vi "HFRR ADV v039 new software.vi"() -> ()   [LabVIEW 2025] (continued)
            n3064 = local read "TITTLE"() -> (w3921:string)
            n3065 = call-poly <vilib>:"Append Report Text.vi"("report in"=w3946, "error in (no error)"=w3945) -> ("report out"=w3967:refnum<class "NI_report.lvclass">, "error out"=w3965:errorcluster)  [unwired: 10 in, 2 out]
            n3066 = Concatenate Strings(w3921, w3920, w3919) -> (→"output":string)
            n3067 = call-poly <vilib>:"Append Report Text.vi"("report in"=w3967, "text"=w3920, "error in (no error)"=w3965) -> ("report out"=w3966:refnum<class "NI_report.lvclass">, "error out"=w3964:errorcluster)  [unwired: 9 in, 2 out]
            n3068 = call-dynamic "Print Report.vi"("report in"=w3966, "printer name (default)"=w3974, "error in (no error)"=w3964) -> ("report out"=w3976:refnum<class "NI_report.lvclass">, "error out"=w3977:errorcluster)  [unwired: 11 in]
            n3069 = call-dynamic "Dispose Report.vi"("report in"=w3976, "error in (no error)"=w3977) -> ()  [unwired: 13 in, 1 out]
          }
        }
      }
    }
    n3070 = case shown="True" "Prog Uno" {
      frame False {
      }
      frame True {
        n3071 = stacked-sequence {
          frame #0 {
            n3072 = Delete(path (use dialog)=path "C:/LAB-IQ-NXT/UNOCOMPILE.bat" ("working directory")) -> ()  [unwired: 4 in, 3 out]
          }
          frame #1 {
            n3073 = local read "Com Port 1"() -> (w2694:refnum<visa-resource-name>)
            n3074 = Concatenate Strings("cmd.exe /c \"mode " ("command line"), w2694, ":1200,n,8,1\"\n" ("command line")) -> (w2699:string)
            n3075 = Concatenate Strings(w2699, "CD\\\nCD WinDucom\navrdude -C avrdude.conf -v -patmega328p -carduino -P" ("command line"), w2694, " -b115200 -D -Uflash:w:UNO_V20.hex:i\n" ("command line"), "\r") -> (w2701:string)
            "STR" <- w2701
            n3076 = call <vilib>:"Write Characters To File.vi"("append to file? (new file:F)"=FALSE, "character string"=w2701, "file path (dialog if empty)"=path "C:/LAB-IQ/UNOCOMPILE.bat" ("working directory")) -> ()  [unwired: 2 in, 1 out]
          }
          frame #2 {
            n3077 = disable-structure shown="Disabled" {
              frame Disabled {
                w2705 = "cmd.exe  /c \"C:\\LAB-IQ-NXT\\UNOCOMPILE.bat\"" ("string")
                n3078 = local write "Prog Uno"(FALSE ("run minimized? (F)")) -> ()
                n3079 = call <vilib>:"System Exec.vi"("expected output size  (4096)"=u32 65535, "run minimized? (F)"=FALSE, "wait until completion? (T)"=TRUE ("run minimized? (F)"), "working directory"=path "C:/LAB-IQ-NXT", "standard input"=w2705, "command line"=w2705) -> ("error out"=w2704:errorcluster, "standard output"=→"String 42":string)  [unwired: 2 in, 2 out]
                "error out 3" <- w2704
                n3080 = flat-sequence {
                  tunnel: w2704 -> [_]
                  frame #0 {
                  }
                }
              }
              frame Enabled {
              }
            }
          }
        }
      }
    }
    n3081 = Wait (ms)(milliseconds to wait=u32 50) -> ()  [unwired: 1 out]
    n3082 = Wait (ms)(milliseconds to wait=u32 50) -> ()  [unwired: 1 out]
    n3083 = local read "Quit"() -> (w2223:bool)
  }
  n3084 = while {
    stop <- w4041 stop-if-true
    n3085 = local read "Auto Start Test"() -> (w4039:bool)
    n3086 = local read "RUN"() -> (w4038:bool)
    n3087 = Wait (ms)(milliseconds to wait=u32 1000) -> ()  [unwired: 1 out]
    n3088 = Or(x=w4038, y=w4039) -> (x .or. y?=w4037:bool)
    n3089 = case shown="True" w4037 {
      frame False {
      }
      frame True {
        n3090 = local read "LVDT STROKE Actual"() -> (w4042:dbl)
        n3091 = In Range and Coerce(upper limit=1.2, x=w4042, lower limit=0.6) -> (In Range?=w4045:bool)  [unwired: 1 out]
        n3092 = call-poly <vilib>:"Random Number (Range).vi"("lower bound (0)"=0.998 ("upper bound (100)"), "upper bound (100)"=1.003) -> ("number"=w4043:dbl)  [unwired: 9 in]
        n3093 = case shown="True" w4045 {
          tunnel: [w4050 w4051] -> w4044
          tunnel: w4043 -> [_ w4051]
          tunnel: w4042 -> [w4050 _]
          frame False {
          }
          frame True {
          }
        }
        "LVDT STROKE DISPLAY" <- w4044
      }
    }
    n3094 = local read "Quit"() -> (w4041:bool)
  }
  n3095 = while {
    tunnel: [w4068] -> w49
    shift-right: [w4061] -> _
    shift-left: 0.0 -> [w4064]
    shift-right: [w4060] -> _
    shift-left: 0.0 -> [w4063]
    shift-right: [w4059] -> _
    shift-left: 100.0 ("vc_cmd") -> [w4062]
    stop <- w4068 stop-if-true
    # "PID LOGIC"
    n3096 = local read "run test Calibration"() -> (w4056:bool)
    n3097 = local read "RUN"() -> (w4066:bool)
    n3098 = local read "Auto Start Temp"() -> (w4057:bool)
    n3099 = local read "Auto Start Test"() -> (w4065:bool)
    n3100 = local read "START TEMP"() -> (w4055:bool)
    n3101 = And(x=w4057, y=w4065) -> (x .and. y?=w4058:bool)
    n3102 = Or(x=w4066, y=w4058) -> (x .or. y?=w4067:bool)
    n3103 = And(x=w4067, y=w4055) -> (x .and. y?=w4054:bool)
    n3104 = And(x=w4056, y=w4055) -> (x .and. y?=w4053:bool)
    n3105 = Or(x=w4053, y=w4054) -> (x .or. y?=w4052:bool)
    n3106 = Wait (ms)(milliseconds to wait="milliseconds to wait") -> ()  [unwired: 1 out]
    n3107 = case shown="True" w4052 {
      tunnel: [400.0 ("out_vc_cmd") w4087] -> w4059
      tunnel: [w4071 w4089] -> w4060
      tunnel: [w4071 w4088] -> w4061
      tunnel: w4064 -> [_ w4078]
      tunnel: w4063 -> [_ w4077]
      tunnel: w4062 -> [_ w4076]
      tunnel: w4056 -> [_ w4072]
      frame False {
        w4071 = 0.0 ("error_out")
      }
      frame True {
        n3108 = case shown="True" w4072 {
          tunnel: [w4096 1.0] -> w4074
          frame False {
            n3109 = local read "Set Strk"() -> (w4095:dbl)
            n3110 = Add(x=w4095, y="Add up Stroke") -> (x+y=w4096:dbl)
          }
          frame True {
          }
        }
        n3111 = local read "LVDT STROKE"() -> (w4073:dbl)
        n3112 = formula code="// Zero-Hardcode Explicit Positional-Form PID Engine\n// Inputs: target_stroke, measured_stroke, dt, prev_error, integral_accumulator_in, prev_vc_cmd\n//         kp, ki, kd, max_step_change, max_amplitude, min_amplitude, startup_cmd\n// Outputs: vc_cmd, error_out, out_error, integral_accumulator_out, out_vc_cmd\n\n// 1. Calculate Tracking Error\nfloat current_error = target_stroke - measured_stroke;\nerror_out = current_error;\n\n// 2. Compute Proportional Term\nfloat p_term = kp * current_error;\n\n// 3. Compute Derivative Term\nfloat d_term = 0.0;\nif (dt > 0.0) {\n    d_term = kd * ((current_error - prev_error) / dt);\n}\n\n// 4. Update and Accumulate Integral Term\nfloat current_integral = integral_accumulator_in + (current_error * dt);\nfloat i_term = ki * current_integral;\n\n// 5. Calculate Ideal Target Command (Anchored by startup baseline)\nfloat ideal_command = startup_cmd + p_term + i_term + d_term;\n\n// 6. Apply Loop Rate Limiting FIRST \n// (Forces the command to climb gradually from prev_vc_cmd instead of jumping straight to max)\nfloat raw_adjustment = ideal_command - prev_vc_cmd;\n\nif (raw_adjustment > max_step_change) {\n    raw_adjustment = max_step_change;\n} else if (raw_adjustment < -max_step_change) {\n    raw_adjustment = -max_step_change;\n}\n\nfloat next_vc_cmd = prev_vc_cmd + raw_adjustment;\n\n// 7. Anti-Windup Protection & Final Output Safety Safeguard Clamping\n// (Back-calculating based on what we are ACTUALLY outputting)\nif (next_vc_cmd > max_amplitude) {\n    float excess = next_vc_cmd - max_amplitude;\n    if (ki > 0.0) {\n        current_integral -= excess / ki;\n    }\n    next_vc_cmd = max_amplitude;\n} else if (next_vc_cmd < min_amplitude) {\n    float excess = next_vc_cmd - min_amplitude;\n    if (ki > 0.0) {\n        current_integral -= excess / ki;\n    }\n    next_vc_cmd = min_amplitude;\n}\n\n// 8. Map to Shift Registers for memory persistence\nvc_cmd = next_vc_cmd;\nout_error = current_error;                   \nintegral_accumulator_out = current_integral;  \nout_vc_cmd = next_vc_cmd;"("target_stroke"=w4074, "measured_stroke"=w4073, "dt"="dt", "integral_accumulator_in"=w4077, "prev_error"=w4078, "prev_vc_cmd"=w4076, "kp"="kp", "ki"="ki", "kd"="kd", "max_step_change"="max_step_change", "max_amplitude"="max_amplitude", "min_amplitude"="min_amplitude", "startup_cmd"="startup_cmd") -> ("vc_cmd"=w4093:dbl, "out_error"=w4088:dbl, "integral_accumulator_out"=w4089:dbl, "out_vc_cmd"=w4087:dbl)  [unwired: 1 out]
        "output Vpp" <- w4093
        n3113 = Number To Fractional String(number=w4093, precision (6)=i16 1) -> (F-format string=w4091:string)  [unwired: 2 in]
        n3114 = Concatenate Strings("DAC;" ("string"), w4091) -> (w4075:string)
        n3115 = local write "Due Write"(w4075) -> ()
        "prev_error" <- w4078
        "integral_accumulator_in" <- w4077
        "prev_vc_cmd" <- w4076
      }
    }
    n3116 = local read "Quit"() -> (w4068:bool)
  }
  n3117 = Or(x=w45, y=w44) -> (x .or. y?=w46:bool)
  n3118 = Or(x=w42, y=w46) -> (x .or. y?=w51:bool)
  n3119 = control-ref of="new picture"() -> ()  [unwired: 1 out]
  n3120 = Or(x=w54, y=w51) -> (x .or. y?=w48:bool)
  n3121 = Or(x=w48, y=w49) -> (x .or. y?=w43:bool)
  n3122 = while {
    tunnel: [w4098] -> w53
    i -> [w4105]
    stop <- w4098 stop-if-true
    n3123 = local read "Quit"() -> (w4098:bool)
    n3124 = Equal To 0?(x=w4105) -> (x = 0?=w4103:bool)
    n3125 = call "Elapsed Time3"("Time Target (s)"=45.0, "Auto Reset"=TRUE) -> ("Time has Elapsed"=w4102:bool)  [unwired: 10 in, 7 out]
    n3126 = Wait (ms)(milliseconds to wait=u32 50) -> ()  [unwired: 1 out]
    n3127 = Or(x=w4102, y=w4103) -> (x .or. y?=w4104:bool)
    n3128 = case shown="True" w4104 {
      frame False {
      }
      frame True {
        n3129 = call <vilib>:"System Exec.vi"("run minimized? (F)"=TRUE, "error in (no error)"="error in (no error)", "command line"="powercfg.exe -change -monitor-timeout-ac 0") -> ("error out"=w4116:errorcluster)  [unwired: 5 in, 3 out]
        n3130 = call <vilib>:"System Exec.vi"("run minimized? (F)"=TRUE, "error in (no error)"=w4116, "command line"="powercfg.exe -change -disk-timeout-ac 0") -> ("error out"=w4115:errorcluster)  [unwired: 5 in, 3 out]
        n3131 = call <vilib>:"System Exec.vi"("run minimized? (F)"=TRUE, "error in (no error)"=w4115, "command line"="powercfg.exe -change -standby-timeout-ac 0") -> ("error out"=w4114:errorcluster)  [unwired: 5 in, 3 out]
        n3132 = call <vilib>:"System Exec.vi"("run minimized? (F)"=TRUE, "error in (no error)"=w4114, "command line"="powercfg.exe -change -hibernate-timeout-ac 0") -> ("error out"=w4113:errorcluster)  [unwired: 5 in, 3 out]
        n3133 = call <vilib>:"Simple Error Handler.vi"("error in (no error)"=w4113) -> ("error out"=w4119:errorcluster)  [unwired: 4 in, 4 out]
        n3134 = call <vilib>:"Clear Errors.vi"("error in (no error)"=w4119) -> ("error out"=→"error out":errorcluster)  [unwired: 5 in, 1 out]
      }
    }
  }
  n3135 = Compound Arithmetic op=OR(w56, w43, w53) -> (w55:bool)
  n3136 = flat-sequence {
    tunnel: w55 -> [_]
    tunnel: [w4121] -> w25
    tunnel: w25 -> [_]
    frame #0 {
      n3137 = call "CLOSE CONNECTION.vi"() -> ("error out"=w4121:errorcluster)  [unwired: 11 in]
    }
    frame #1 {
      n3138 = Quit LabVIEW(quit? (T)=TRUE) -> ()
      n3139 = local write "Quit"(FALSE ("EXIT")) -> ()
    }
  }
  n3140 = property on="Heater Button" class="Bool (strict)"("Visible"=TRUE) -> ()  [unwired: 2 in, 2 out]
  n3141 = while {
    tunnel: [w4128] -> _
    i -> [w4128]
    stop <- w4124 stop-if-true
    # "Langauage selection"
    n3142 = Equal?(x="Lan flag", y=22.0) -> ()  [unwired: 1 out]
    n3143 = disable-structure shown="Disabled" {
      frame Disabled {
        n3144 = stacked-sequence {
          frame #0 {
            n3145 = case shown="\"Russian\"" "Language Selection" {
              tunnel: [0 1] -> w4130
              frame "English", Default {
              }
              frame "Russian" {
              }
            }
            n3146 = for {
              N: 130 -> [_]
              tunnel: "Table" -> [w4139]
              tunnel: w4130 -> [w4138]
              i -> [w4137]
              n3147 = Index Array(array=w4139, index (row)=w4137, index (col)=w4138) -> (element=w4136:string)
              n3148 = case shown="1" w4137 {
                tunnel: w4136 -> [w4140 w4141 _ w4142 w4143 w4144 w4145 w4146 w4147 w4148 w4149 w4150 w4151 w4152 w4153 w4154 w4155 w4156 w4157 w4158 w4159 w4160 w4161 w4162 w4163 w4164 w4165 w4166 w4167 _ _ w4168 w4169 w4170 w4171 w4172 w4173 w4182 w4189 w4196 w4203 w4207 w4210 w4213 w4215 w4217 w4218 w4219 w4220 w4221 w4222 w4223 w4224 w4225 w4226 w4227 w4228 w4229 w4230 w4231 w4232 w4233 w4234 w4235 w4236 w4237 w4238 w4239 w4240 w4241 w4242 w4243 w4244 w4245 w4246 w4247 w4248 w4249 w4250 w4251 w4252 w4253 w4254 w4255 w4256 w4257 w4258 w4259 w4260 w4261 w4262 w4263 w4264 w4265 w4266 w4267 w4268 w4269 w4270 w4271 w4272 w4273 w4274 w4275 w4276 _ w4277 w4278 w4279 w4280 w4281 w4282 w4283 w4284 w4285 w4286 w4287 w4288 w4289 _ w4290 w4291 w4292 w4293 w4294 w4295 _]
                frame 0 {
                  n3149 = local write "S"(w4140) -> ()
                }
                frame 1 {
                  n3150 = local write "S 2"(w4141) -> ()
                }
                frame 2 {
                }
                frame 3 {
                  n3151 = local write "S 4"(w4142) -> ()
                }
                frame 4 {
                  n3152 = property on="FILE" class="Str"("Caption.Text"=w4143) -> ()  [unwired: 2 in, 2 out]
                }
                frame 5 {
                  n3153 = property on="Fuel Discription :" class="Str"("Caption.Text"=w4144) -> ()  [unwired: 2 in, 2 out]
                }
                frame 6 {
                  n3154 = property on="Remarks :" class="Str"("Caption.Text"=w4145) -> ()  [unwired: 2 in, 2 out]
                }
                frame 7 {
                  n3155 = property on="Save & Continue" class="Bool (strict)"("Boolean Text.Text"=w4146) -> ()  [unwired: 2 in, 2 out]
                }
                frame 8 {
                }
                frame 9 {
                  n3156 = property on="Set Hz" class="DigNum (strict)"("Caption.Text"=w4148) -> ()  [unwired: 2 in, 2 out]
                }
                frame 10 {
                }
                frame 11 {
                  n3157 = property on="NORMAL LOAD" class="DigNum (strict)"("Caption.Text"=w4150) -> ()  [unwired: 2 in, 2 out]
                }
                frame 12 {
                }
                frame 13 {
                  n3158 = property on="Set Temp" class="DigNum (strict)"("Caption.Text"=w4152) -> ()  [unwired: 2 in, 2 out]
                }
                frame 14 {
                  n3159 = local write "S 15"(w4153) -> ()
                }
                frame 15 {
                  n3160 = property on="Set Rh" class="DigNum (strict)"("Caption.Text"=w4154) -> ()  [unwired: 2 in, 2 out]
                }
                frame 16 {
                }
                frame 17 {
                  n3161 = local write "S 18"(w4156) -> ()
                }
                frame 18 {
                  "String 17" <- w4157
                }
                frame 19 {
                  n3162 = property on="test time" class="DigNum (strict)"("Caption.Text"=w4158) -> ()  [unwired: 2 in, 2 out]
                }
                frame 20 {
                  "String 18" <- w4159
                  "String 22" <- w4159
                }
                frame 21 {
                  n3163 = property on="Elapsed time" class="DigNum (strict)"("Caption.Text"=w4160) -> ()  [unwired: 2 in, 2 out]
                }
                frame 22 {
                  n3164 = property on="Samplingtime 2" class="DigNum (strict)"("Caption.Text"=w4161) -> ()  [unwired: 2 in, 2 out]
                }
                frame 23 {
                  "String 21" <- w4162
                }
                frame 24 {
                  n3165 = property on="Countdown" class="DigNum (strict)"("Caption.Text"=w4163) -> ()  [unwired: 2 in, 2 out]
                }
                frame 25 {
                  n3166 = property on="Countdown 2" class="DigNum (strict)"("Caption.Text"=w4164) -> ()  [unwired: 2 in, 2 out]
                }
                frame 26 {
                  n3167 = property on="Engage" class="Bool (strict)"("Boolean Text.Text"=w4165) -> ()  [unwired: 2 in, 2 out]
                }
                frame 27 {
                  n3168 = property on="Boolean  4" class="Bool (strict)"("Boolean Text.Text"=w4166) -> ()  [unwired: 2 in, 2 out]
                }
                frame 28 {
                  n3169 = property on="Test \nStatus" class="Bool (strict)"("Boolean Text.Text"=w4167) -> ()  [unwired: 2 in, 2 out]
                }
                frame 29 {
                }
                frame 30 {
                }
                frame 31 {
                }
                frame 32 {
                  n3170 = property on="RSTCOF" class="Bool"("Boolean Text.Text"=w4169) -> ()  [unwired: 2 in, 2 out]
                  n3171 = property on="RST FF" class="Bool"("Boolean Text.Text"=w4169) -> ()  [unwired: 2 in, 2 out]
                  n3172 = property on="RST TEMP" class="Bool"("Boolean Text.Text"=w4169) -> ()  [unwired: 2 in, 2 out]
                  n3173 = property on="RSTV1 3" class="Bool"("Boolean Text.Text"=w4169) -> ()  [unwired: 2 in, 2 out]
                  n3174 = property on="rstv2" class="Bool"("Boolean Text.Text"=w4169) -> ()  [unwired: 2 in, 2 out]
                  n3175 = property on="RSTV1 2" class="Bool"("Boolean Text.Text"=w4169) -> ()  [unwired: 2 in, 2 out]
                  n3176 = property on="RST CP" class="Bool"("Boolean Text.Text"=w4169) -> ()  [unwired: 2 in, 2 out]
                }
                frame 33 {
                  "S 61" <- w4170
                }
                frame 34 {
                  "String 23" <- w4171
                }
                frame 35 {
                  n3177 = property on="Rh Before" class="DigNum (strict)"("Caption.Text"=w4172) -> ()  [unwired: 2 in, 2 out]
                }
                frame 36 {
                  n3178 = Match Pattern(string=w4173, regular expression=",") -> (before substring=→"bs":string, after substring=→"as":string)  [unwired: 1 in, 2 out]
                  n3179 = property on="Rh After" class="DigNum (strict)"("Caption.Text"=w4173) -> ()  [unwired: 2 in, 2 out]
                }
                frame 37 {
                  n3180 = Match Pattern(string=w4182, regular expression=",") -> (before substring=w4181:string, after substring=w4180:string)  [unwired: 1 in, 2 out]
                  "bs" <- w4181
                  "as" <- w4180
                  n3181 = Concatenate Strings(w4181, w4180) -> (w4177:string)
                  n3182 = property on="Humidity before test 2" class="DigNum (strict)"("Caption.Text"=w4177) -> ()  [unwired: 2 in, 2 out]
                  n3183 = Concatenate Strings(w4177, "=" ("string")) -> (w4178:string)
                  n3184 = local write "S 38"(w4178) -> ()
                }
                frame 38 {
                  n3185 = Match Pattern(string=w4189, regular expression=",") -> (before substring=w4188:string, after substring=w4187:string)  [unwired: 1 in, 2 out]
                  "bs" <- w4188
                  "as" <- w4187
                  n3186 = Concatenate Strings(w4188, w4187) -> (w4184:string)
                  n3187 = property on="Humidity after test 2" class="DigNum (strict)"("Caption.Text"=w4184) -> ()  [unwired: 2 in, 2 out]
                  n3188 = Concatenate Strings(w4184, "=" ("string")) -> (w4186:string)
                  n3189 = local write "S 39"(w4186) -> ()
                }
                frame 39 {
                  n3190 = Match Pattern(string=w4196, regular expression=",") -> (before substring=w4195:string, after substring=w4194:string)  [unwired: 1 in, 2 out]
                  "bs" <- w4195
                  "as" <- w4194
                  n3191 = Concatenate Strings(w4195, w4194) -> (w4191:string)
                  n3192 = property on="Temperature before test 2" class="DigNum (strict)"("Caption.Text"=w4191) -> ()  [unwired: 2 in, 2 out]
                  n3193 = Concatenate Strings(w4191, "=" ("string")) -> (→"String 34":string)
                }
                frame 40 {
                  n3194 = Match Pattern(string=w4203, regular expression=",") -> (before substring=w4202:string, after substring=w4201:string)  [unwired: 1 in, 2 out]
                  "bs" <- w4202
                  "as" <- w4201
                  n3195 = Concatenate Strings(w4202, w4201) -> (w4198:string)
                  n3196 = property on="Temperature after test 2" class="DigNum (strict)"("Caption.Text"=w4198) -> ()  [unwired: 2 in, 2 out]
                  n3197 = Concatenate Strings(w4198, "=" ("string")) -> (→"String 35":string)
                  n3198 = property on="Temperature after test" class="DigNum (strict)"("Caption.Text"=w4198) -> ()  [unwired: 2 in, 2 out]
                }
                frame 41 {
                  n3199 = property on="AVP 2" class="DigNum (strict)"("Caption.Text"=w4207) -> ()  [unwired: 2 in, 2 out]
                  n3200 = Concatenate Strings(w4207, "=" ("string")) -> (→"String 36":string)
                }
                frame 42 {
                  n3201 = property on="MWSD 2" class="DigNum (strict)"("Caption.Text"=w4210) -> ()  [unwired: 2 in, 2 out]
                  n3202 = Concatenate Strings(w4210, "=" ("string")) -> (→"String 37":string)
                }
                frame 43 {
                  n3203 = property on="HCF 2" class="DigNum (strict)"("Caption.Text"=w4213) -> ()  [unwired: 2 in, 2 out]
                  n3204 = Concatenate Strings(w4213, "=" ("string")) -> (→"String 38":string)
                }
                frame 44 {
                  n3205 = Concatenate Strings(w4215, "=" ("string")) -> (→"String 39":string)
                  n3206 = property on="WS1.4 2" class="DigNum (strict)"("Caption.Text"=w4215) -> ()  [unwired: 2 in, 2 out]
                }
                frame 45 {
                }
                frame 46 {
                  n3207 = local write "S 47"(w4218) -> ()
                }
                frame 47 {
                  n3208 = local write "S 48"(w4219) -> ()
                }
                frame 48 {
                  n3209 = local write "S 49"(w4220) -> ()
                }
                frame 49 {
                  n3210 = local write "S 50"(w4221) -> ()
                }
                frame 50 {
                  n3211 = local write "S 51"(w4222) -> ()
                }
                frame 51 {
                  n3212 = local write "S 52"(w4223) -> ()
                }
                frame 52 {
                  n3213 = local write "S 53"(w4224) -> ()
                }
                frame 53 {
                  n3214 = local write "S 54"(w4225) -> ()
                }
                frame 54 {
                  n3215 = local write "S 55"(w4226) -> ()
                }
                frame 55 {
                  n3216 = local write "S 56"(w4227) -> ()
                }
                frame 56 {
                  n3217 = local write "S 57"(w4228) -> ()
                }
                frame 57 {
                  n3218 = local write "S 58"(w4229) -> ()
                }
                frame 58 {
                  n3219 = local write "S 59"(w4230) -> ()
                }
                frame 59 {
                  n3220 = local write "S 60"(w4231) -> ()
                }
                frame 60 {
                  n3221 = local write "S 62"(w4232) -> ()
                }
                frame 61 {
                  n3222 = local write "S 63"(w4233) -> ()
                }
                frame 62 {
                  n3223 = local write "S 64"(w4234) -> ()
                }
                frame 63 {
                  n3224 = local write "S 65"(w4235) -> ()
                }
                frame 64 {
                  n3225 = local write "S 66"(w4236) -> ()
                }
                frame 65 {
                  n3226 = local write "S 67"(w4237) -> ()
                }
                frame 66 {
                  n3227 = local write "S 68"(w4238) -> ()
                }
                frame 67 {
                  n3228 = local write "S 69"(w4239) -> ()
                }
                frame 68 {
                  n3229 = local write "S 70"(w4240) -> ()
                }
                frame 69 {
                  n3230 = local write "S 71"(w4241) -> ()
                }
                frame 70 {
                  n3231 = local write "S 72"(w4242) -> ()
                }
                frame 71 {
                  n3232 = local write "S 73"(w4243) -> ()
                }
                frame 72 {
                  n3233 = local write "S 74"(w4244) -> ()
                }
                frame 73 {
                  n3234 = local write "S 75"(w4245) -> ()
                }
                frame 74 {
                  n3235 = local write "S 76"(w4246) -> ()
                }
                frame 75 {
                  n3236 = local write "S 77"(w4247) -> ()
                }
                frame 76 {
                  n3237 = local write "S 78"(w4248) -> ()
                }
                frame 77 {
                  n3238 = local write "S 79"(w4249) -> ()
                }
                frame 79 {
                  n3239 = property on="Sample Temperature ( °C )" class="XYGraph (strict)"("Y Scale.Name Label.Text"=w4250) -> ()  [unwired: 2 in, 2 out]
                }
                frame 80 {
                  n3240 = local write "S 81"(w4251) -> ()
                  n3241 = property on="Humidity ( %RH )" class="XYGraph (strict)"("Y Scale.Name Label.Text"=w4251) -> ()  [unwired: 2 in, 2 out]
                }
                frame 78 {
                  n3242 = property on="Air Temperature  ( °C )" class="XYGraph (strict)"("X Scale.Name Label.Text"=w4252) -> ()  [unwired: 2 in, 2 out]
                  n3243 = property on="Humidity ( %RH )" class="XYGraph (strict)"("X Scale.Name Label.Text"=w4252) -> ()  [unwired: 2 in, 2 out]
                  n3244 = property on="Sample Temperature ( °C )" class="XYGraph (strict)"("X Scale.Name Label.Text"=w4252) -> ()  [unwired: 2 in, 2 out]
                  n3245 = property on="Coefficient Of Friction" class="XYGraph (strict)"("X Scale.Name Label.Text"=w4252) -> ()  [unwired: 2 in, 2 out]
                }
                frame 81 {
                  n3246 = property on="Air Temperature  ( °C )" class="XYGraph (strict)"("Y Scale.Name Label.Text"=w4253) -> ()  [unwired: 2 in, 2 out]
                }
                frame 82 {
                  n3247 = local write "S 84"(w4254) -> ()
                }
                frame 83 {
                  n3248 = local write "S 85"(w4255) -> ()
                }
                frame 84 {
                  n3249 = local write "S 86"(w4256) -> ()
                }
                frame 85 {
                  n3250 = local write "S 87"(w4257) -> ()
                }
                frame 86 {
                  n3251 = local write "S 88"(w4258) -> ()
                }
                frame 87 {
                }
                frame 88 {
                  n3252 = local write "S 90"(w4260) -> ()
                }
                frame 89 {
                  n3253 = local write "S 91"(w4261) -> ()
                }
                frame 90 {
                  n3254 = local write "S 92"(w4262) -> ()
                }
                frame 91 {
                  n3255 = local write "S 93"(w4263) -> ()
                }
                frame 92 {
                  n3256 = local write "S 94"(w4264) -> ()
                }
                frame 93 {
                  n3257 = local write "S 95"(w4265) -> ()
                }
                frame 94 {
                  n3258 = local write "S 96"(w4266) -> ()
                }
                frame 95 {
                  n3259 = local write "S 97"(w4267) -> ()
                }
                frame 96 {
                  n3260 = local write "S 98"(w4268) -> ()
                }
                frame 97 {
                  n3261 = local write "S 99"(w4269) -> ()
                }
                frame 98 {
                  n3262 = local write "S 100"(w4270) -> ()
                }
                frame 99 {
                  n3263 = local write "S 101"(w4271) -> ()
                }
                frame 100 {
                  n3264 = local write "S 102"(w4272) -> ()
                }
                frame 101 {
                  n3265 = local write "S 103"(w4273) -> ()
                }
                frame 102 {
                  n3266 = local write "S 104"(w4274) -> ()
                }
                frame 103 {
                  n3267 = local write "S 105"(w4275) -> ()
                }
                frame 104 {
                  n3268 = local write "S 106"(w4276) -> ()
                }
                frame 105 {
                }
                frame 106 {
                  n3269 = property on="OK Button 17" class="Bool (strict)"("Boolean Text.Text"=w4277) -> ()  [unwired: 2 in, 2 out]
                }
                frame 107 {
                  n3270 = property on="OK Button 16" class="Bool (strict)"("Boolean Text.Text"=w4278) -> ()  [unwired: 2 in, 2 out]
                }
                frame 108 {
                  n3271 = property on="TITTLE" class="Str"("Caption.Text"=w4279) -> ()  [unwired: 2 in, 2 out]
                }
                frame 109 {
                  "String 30" <- w4280
                }
                frame 110 {
                  n3272 = property on="Test Date" class="Str"("Caption.Text"=w4281) -> ()  [unwired: 2 in, 2 out]
                  "String 31" <- w4281
                }
                frame 111 {
                  n3273 = property on="Sample ID" class="Str"("Caption.Text"=w4282) -> ()  [unwired: 2 in, 2 out]
                  "String 32" <- w4282
                }
                frame 112 {
                  n3274 = property on="Tested by" class="Str"("Caption.Text"=w4283) -> ()  [unwired: 2 in, 2 out]
                  "String 33" <- w4283
                }
                frame 113 {
                  n3275 = property on="System Configured Printers 2" class="Arr (strict)"("Caption.Text"=w4284) -> ()  [unwired: 2 in, 2 out]
                }
                frame 114 {
                  n3276 = property on="Selected Printer" class="Str"("Caption.Text"=w4285) -> ()  [unwired: 2 in, 2 out]
                }
                frame 115 {
                  n3277 = property on="Select Printer 3" class="DigNum (strict)"("Caption.Text"=w4286) -> ()  [unwired: 2 in, 2 out]
                }
                frame 116 {
                  n3278 = property on="Print" class="Bool (strict)"("Boolean Text.Text"=w4287) -> ()  [unwired: 2 in, 2 out]
                }
                frame 117 {
                  "String 41" <- w4288
                }
                frame 118 {
                  n3279 = property on="tested by" class="Str"("Caption.Text"=w4289) -> ()  [unwired: 2 in, 2 out]
                }
                frame 119 {
                }
                frame 120 {
                  n3280 = property on="Export" class="Bool (strict)"("Boolean Text.Text"=w4290) -> ()  [unwired: 2 in, 2 out]
                }
                frame 121 {
                }
                frame 122 {
                }
                frame 123 {
                  n3281 = property on="Select File Type" class="Enum (strict)"("Caption.Text"=w4293) -> ()  [unwired: 2 in, 2 out]
                }
                frame 124 {
                  n3282 = property on="s.NO" class="Str"("Caption.Text"=w4294) -> ()  [unwired: 2 in, 2 out]
                  "String 45" <- w4294
                }
                frame 125 {
                  n3283 = property on="trip1 8" class="Bool (strict)"("Boolean Text.Text"=w4295) -> ()  [unwired: 2 in, 2 out]
                }
                frame 126, Default {
                }
              }
            }
          }
          frame #1 {
            w4303 = TRUE ("Visible")
            n3284 = local read "S 91"() -> (w4320:string)
            n3285 = local read "S 90"() -> (w4319:string)
            n3286 = local read "S 88"() -> (w4318:string)
            n3287 = property on="File Path" class="Path"("Caption.Text"=w4319) -> ()  [unwired: 2 in, 2 out]
            n3288 = local read "S 71"() -> (w4313:string)
            n3289 = local read "S 86"() -> (w4315:string)
            n3290 = local read "S 85"() -> (w4316:string)
            n3291 = local read "S 87"() -> (w4314:string)
            n3292 = local read "S 84"() -> (w4317:string)
            n3293 = local read "S 103"() -> (w4302:string)
            n3294 = local read "S 104"() -> (w4301:string)
            n3295 = property on="Password" class="Str"("Caption.Text"=w4316) -> ()  [unwired: 2 in, 2 out]
            n3296 = property on="EDIT" class="Bool (strict)"("Boolean Text.Text"=w4313) -> ()  [unwired: 2 in, 2 out]
            n3297 = property on="SAVE" class="Bool (strict)"("Boolean Text.Text"=w4317) -> ()  [unwired: 2 in, 2 out]
            n3298 = Build Array(w4302, w4301) -> (w4300:string[])
            n3299 = property on="Heater Button" class="Bool (strict)"("Strings [4]"=w4300) -> ()  [unwired: 2 in, 2 out]
            n3300 = local read "S 92"() -> (w4312:string)
            n3301 = local read "S 93"() -> (w4311:string)
            n3302 = local read "S 105"() -> (w4298:string)
            n3303 = local read "S 106"() -> (w4297:string)
            n3304 = Build Array(w4312, w4311) -> ()  [unwired: 1 out]
            n3305 = Build Array(w4298, w4297) -> (w4299:string[])
            n3306 = local read "S 95"() -> (w4309:string)
            n3307 = local read "S 94"() -> (w4310:string)
            n3308 = local read "bs"() -> (w4325:string)
            n3309 = local read "as"() -> (w4326:string)
            n3310 = property on="Humidity" class="Bool (strict)"("Strings [4]"=w4299) -> ()  [unwired: 2 in, 2 out]
            n3311 = Concatenate Strings(w4325, "\r", w4326) -> ()  [unwired: 1 out]
            n3312 = property on="Rh After" class="DigNum (strict)"("Caption.Size to Text?"=TRUE ("Caption.Size to Text")) -> ()  [unwired: 2 in, 2 out]
            n3313 = local read "S 48"() -> (w4349:string)
            n3314 = local read "S 50"() -> (w4347:string)
            n3315 = local read "S 51"() -> (w4346:string)
            n3316 = local read "S 49"() -> (w4348:string)
            n3317 = local read "S 52"() -> (w4345:string)
            n3318 = local read "as"() -> (w4330:string)
            n3319 = local read "bs"() -> (w4331:string)
            n3320 = local read "S 56"() -> (w4344:string)
            n3321 = local read "S 57"() -> (w4343:string)
            n3322 = local read "S 58"() -> (w4342:string)
            n3323 = local read "S 59"() -> (w4341:string)
            n3324 = property on="OPEN" class="Bool (strict)"("Boolean Text.Text"=w4345) -> ()  [unwired: 2 in, 2 out]
            n3325 = property on="OPEN 1" class="Bool (strict)"("Boolean Text.Text"=w4349) -> ()  [unwired: 2 in, 2 out]
            n3326 = property on="OPEN 2" class="Bool (strict)"("Boolean Text.Text"=w4348) -> ()  [unwired: 2 in, 2 out]
            n3327 = property on="OPEN 3" class="Bool (strict)"("Boolean Text.Text"=w4347) -> ()  [unwired: 2 in, 2 out]
            n3328 = property on="OPEN 4" class="Bool (strict)"("Boolean Text.Text"=w4346) -> ()  [unwired: 2 in, 2 out]
            n3329 = Concatenate Strings(w4331, "\r", w4330) -> ()  [unwired: 1 out]
            n3330 = local read "S 102"() -> (w4304:string)
            n3331 = property on="КОФ1" class="DigNum (strict)"("Caption.Text"=w4344) -> ()  [unwired: 2 in, 2 out]
            n3332 = local read "S 98"() -> (w4308:string)
            n3333 = local read "S 99"() -> (w4307:string)
            n3334 = local read "S 100"() -> (w4306:string)
            n3335 = local read "S 101"() -> (w4305:string)
            n3336 = property on="КОФ2" class="DigNum (strict)"("Caption.Text"=w4343) -> ()  [unwired: 2 in, 2 out]
            n3337 = property on="КОФ3" class="DigNum (strict)"("Caption.Text"=w4342) -> ()  [unwired: 2 in, 2 out]
            n3338 = property on="КОФ4" class="DigNum (strict)"("Caption.Text"=w4341) -> ()  [unwired: 2 in, 2 out]
            n3339 = local read "bs"() -> (w4329:string)
            n3340 = local read "as"() -> (w4328:string)
            n3341 = local read "S 60"() -> (w4340:string)
            n3342 = local read "S 54"() -> (w4350:string)
            n3343 = Concatenate Strings(w4329, "\r", w4328) -> ()  [unwired: 1 out]
            n3344 = Concatenate Strings(w4350, w4340) -> ()  [unwired: 1 out]
            n3345 = local read "S 77"() -> (→"String 43":string)
            n3346 = local read "S 76"() -> (w4323:string)
            n3347 = local read "S 78"() -> (w4322:string)
            n3348 = local read "S 71"() -> (w4334:string)
            n3349 = local read "S 66"() -> (w4339:string)
            n3350 = local read "S 67"() -> (w4338:string)
            n3351 = local read "S 68"() -> (w4337:string)
            n3352 = local read "S 69"() -> (w4336:string)
            n3353 = local read "S 70"() -> (w4335:string)
            n3354 = property on="AIR TEMP" class="DigNum (strict)"("Caption.Text"=w4322) -> ()  [unwired: 2 in, 2 out]
            n3355 = property on="Set Strk" class="DigNum (strict)"("Caption.Text"=w4323) -> ()  [unwired: 2 in, 2 out]
            n3356 = property on="SPEED OUT:" class="DigNum (strict)"("Caption.Text"=w4337) -> ()  [unwired: 2 in, 2 out]
            n3357 = property on="EDIT" class="Bool (strict)"("Boolean Text.Text"=w4334) -> ()  [unwired: 2 in, 2 out]
            n3358 = local read "S 79"() -> (w4321:string)
          }
          frame #2 {
          }
        }
        n3359 = local write "Lan flag"(10.0 ("Lan flag")) -> ()
      }
      frame Enabled {
      }
    }
    n3360 = Wait (ms)(milliseconds to wait=u32 2000) -> ()  [unwired: 1 out]
    n3361 = local read "Quit"() -> (w4124:bool)
  }
  n3362 = while {
    shift-right: [w4356] -> _
    shift-left: _ -> [w4357]
    shift-right: [w4354] -> _
    shift-left: T18 {"Read Heave and Surge"="", "Bytes at Heave Port"=0.0, "Heave and Surge COM Port:"="COM9", "Com Port 2"="COM7", "Residual Due"="", "Heave COM Status 2"=TRUE, "Heave COM Status"=TRUE, "Port 2"=TRUE, "Sway PPR"=6400.0, "Surge PPR"=6400.0, "Heave PPR"=6400.0, "Sway Pitch"=2.0, "Surge Pitch"=3.0, "Heave Pitch"=4.0, "Sway Pulses/mm"=320.0, "Surge Pulses/mm"=1600.0, "Heave Pulses/mm"=1600.0, "inner loop"=0.0, "Read Heave and Surge 2"="", "String 36"="", "Write S"=FALSE, "WriteCC1"=[""], "Heave COM Loop"=0, "LastCom"="", "EXIT"=FALSE, "Error Heave"={"status"=TRUE, "code"=-1073807343, "source"=""}} -> [w4353]
    shift-right: [w4351] -> _
    shift-left: enum16{"init", "MAIN", "Panel Close"}."init" -> [w4352]
    stop <- w4355 stop-if-true
    # "HUMIDITY LOOP LOGIC"
    n3363 = case shown="\"MAIN\"" w4352 {
      tunnel: w4357 -> [w4371 w4395 w4459 w4461]
      tunnel: [w4366 w4382 w4459 w4461] -> w4356
      tunnel: [_ _ TRUE _] -> w4355
      tunnel: [w4363 w4380 w4457 w4460] -> w4354
      tunnel: w4353 -> [w4368 w4394 w4457 w4460]
      tunnel: [enum16{"init", "MAIN", "Panel Close"}."MAIN" w4389 _ _] -> w4351
      frame "init" {
        n3364 = local read "C3 :"() -> (w4358:refnum<visa-resource-name>)
        n3365 = Bundle By Name(cluster=w4368, "Heave and Surge COM Port:"=w4358) -> (w4367:T18)
        n3366 = call "Instrument fgv uno.vi"("Enum"=T32."INIT", "error in (no error) 2"=w4371, "INPUT"=w4367) -> ("error"=w4369:errorcluster, "output"=w4365:T18)  [unwired: 6 in, 1 out]
        n3367 = case shown="Error" w4369 {
          selector: w4369 -> [w4373 _]
          tunnel: [w4373 w4377] -> w4366
          tunnel: w4365 -> [w4372 w4375]
          tunnel: [w4372 w4374] -> w4364
          frame No Error {
          }
          frame Error {
            n3368 = call "Instrument fgv uno.vi"("Enum"=T32."ERROR INIT", "INPUT"=w4375) -> ("error"=w4378:errorcluster, "output"=w4374:T18)  [unwired: 7 in, 1 out]
            n3369 = call <vilib>:"Clear Errors.vi"("error in (no error)"=w4378) -> ("error out"=w4377:errorcluster)  [unwired: 5 in, 1 out]
          }
        }
        n3370 = local read "LastCom Humidity"() -> (w4361:string)
        n3371 = Unbundle By Name(w4364) -> ("Heave COM Status 2"=→"COM Status":bool, "Error Heave"=→"Error":errorcluster)  [unwired: 1 out]
        n3372 = Bundle By Name(cluster=w4364, "LastCom"=w4361) -> (w4363:T18)
      }
      frame "MAIN" {
        n3373 = Unbundle By Name(w4394) -> ("Com Port 2"=w4384:refnum<visa-resource-name>)
        n3374 = local read "C3 :"() -> (w4385:refnum<visa-resource-name>)
        n3375 = local write "COM Port Humidity :"(w4384) -> ()
        n3376 = Bundle By Name(cluster=w4394, "Heave and Surge COM Port:"=w4385) -> (w4393:T18)
        n3377 = Equal?(x=w4384, y=w4385) -> (x = y?=w4398:bool)
        n3378 = case shown="False" w4398 {
          tunnel: [w4413 w4430] -> w4383
          tunnel: w4395 -> [w4414 w4436]
          tunnel: w4393 -> [w4412 w4434]
          tunnel: [w4411 w4429] -> w4381
          frame False {
            n3379 = call <vilib>:"Clear Errors.vi"("error in (no error)"=w4414) -> ("error out"=w4410:errorcluster)  [unwired: 5 in, 1 out]
            n3380 = call "Instrument fgv uno.vi"("Enum"=T32."ERROR INIT", "error in (no error) 2"=w4410, "INPUT"=w4412) -> ("error"=w4416:errorcluster, "output"=w4411:T18)  [unwired: 6 in, 1 out]
            n3381 = call <vilib>:"Clear Errors.vi"("error in (no error)"=w4416) -> ("error out"=w4413:errorcluster)  [unwired: 5 in, 1 out]
          }
          frame True {
            n3382 = call "Instrument fgv uno.vi"("Enum"=T32."READ", "error in (no error) 2"=w4436, "INPUT"=w4434) -> ("error"=w4435:errorcluster, "output"=w4428:T18)  [unwired: 6 in, 1 out]
            n3383 = Bundle By Name(cluster=w4428, "String 36"="WRITE HUMIDITY") -> (w4427:T18)
            n3384 = case shown="True" "Write Humidity" {
              selector: "Write Humidity" -> [_ w4456]
              tunnel: w4435 -> [w4449 w4455]
              tunnel: [w4449 w4454] -> w4425
              tunnel: w4427 -> [w4448 w4452]
              tunnel: [w4448 w4451] -> w4424
              frame False {
              }
              frame True {
                n3385 = Not(x=w4456) -> (.not. x?=w4450:bool)
                n3386 = local write "Write Humidity"(w4450) -> ()
                n3387 = call "Instrument fgv uno.vi"("Enum"=T32."MANUAL WRITE", "error in (no error) 2"=w4455, "INPUT"=w4452) -> ("error"=w4454:errorcluster, "output"=w4451:T18)  [unwired: 6 in, 1 out]
              }
            }
            n3388 = Array Size(array="WriteHumidity") -> (size(s)=w4422:i32)
            n3389 = Greater Than 0?(x=w4422) -> (x > 0?=w4421:bool)
            n3390 = call "Instrument fgv uno.vi"("Enum"=T32."WRITE", "error in (no error) 2"=w4425, "WriteCC1"="WriteHumidity", "INPUT"=w4424) -> ("error"=w4432:errorcluster, "WriteCC1 2"=w4423:string[], "output"=w4431:T18)  [unwired: 5 in]
            n3391 = case shown="True" w4421 {
              tunnel: w4423 -> [_ w4438]
              frame False {
              }
              frame True {
                n3392 = local write "WriteHumidity"(w4438) -> ()
              }
            }
            n3393 = case shown="No Error" w4432 {
              selector: w4432 -> [w4439 w4442]
              tunnel: w4431 -> [w4440 w4447]
              tunnel: [w4440 w4446] -> w4429
              tunnel: [w4439 w4444] -> w4430
              frame No Error {
              }
              frame Error {
                n3394 = call <vilib>:"Clear Errors.vi"("error in (no error)"=w4442) -> ("error out"=w4441:errorcluster)  [unwired: 5 in, 1 out]
                n3395 = call "Instrument fgv uno.vi"("Enum"=T32."ERROR INIT", "error in (no error) 2"=w4441, "INPUT"=w4447) -> ("error"=w4445:errorcluster, "output"=w4446:T18)  [unwired: 6 in, 1 out]
                n3396 = call <vilib>:"Clear Errors.vi"("error in (no error)"=w4445) -> ("error out"=w4444:errorcluster)  [unwired: 5 in, 1 out]
              }
            }
            n3397 = Unbundle By Name(w4429) -> ("LastCom"=→"LastCom Humidity":string, "Read Heave and Surge"=→"Read HUMIDITY":string)
          }
        }
        n3398 = Unbundle By Name(w4381) -> ("Heave COM Status 2"=w4397:bool, "Error Heave"=w4386:errorcluster, "Bytes at Heave Port"=→"Bytes at Humidity Port  2":dbl)  [unwired: 1 out]
        n3399 = Unbundle By Name(w4386) -> ("status"=→"Humidity Port":bool)
        n3400 = Not(x=w4397) -> (.not. x?=w4387:bool)
        n3401 = local write "Error"(w4386) -> ()
        n3402 = local read "HUMIDITY CLEAR"() -> (w4379:bool)
        n3403 = local read "Quit"() -> (w4390:bool)
        n3404 = local write "COM Status"(w4387) -> ()
        n3405 = Select(t=enum16{"init", "MAIN", "Panel Close"}."Panel Close", s=w4390, f=enum16{"init", "MAIN", "Panel Close"}."MAIN") -> (s? t:f=w4389:enum16{"init", "MAIN", "Panel Close"})
        n3406 = case shown="True" w4379 {
          selector: w4379 -> [_ w4402]
          tunnel: w4383 -> [w4400 w4406]
          tunnel: [w4400 w4405] -> w4382
          tunnel: w4381 -> [w4399 w4404]
          tunnel: [w4399 w4403] -> w4380
          frame False {
          }
          frame True {
            n3407 = Not(x=w4402) -> (.not. x?=w4401:bool)
            n3408 = local write "HUMIDITY CLEAR"(w4401) -> ()
            n3409 = call <vilib>:"Clear Errors.vi"("error in (no error)"=w4406) -> ("error out"=w4408:errorcluster)  [unwired: 5 in, 1 out]
            n3410 = call "Instrument fgv uno.vi"("Enum"=T32."ERROR INIT", "error in (no error) 2"=w4408, "INPUT"=w4404) -> ("error"=w4409:errorcluster, "output"=w4403:T18)  [unwired: 6 in, 1 out]
            n3411 = call <vilib>:"Clear Errors.vi"("error in (no error)"=w4409) -> ("error out"=w4405:errorcluster)  [unwired: 5 in, 1 out]
          }
        }
      }
      frame "Panel Close" {
      }
      frame Default {
      }
    }
  }
  n3412 = while {
    stop <- w4464 stop-if-true
    n3413 = call <vilib>:"High Resolution Polling Wait.vi"("seconds to wait"=0.05) -> ()  [unwired: 10 in, 1 out]
    n3414 = disable-structure shown="Disabled" {
      disable-tunnel: [_ w4495] -> w4462
      frame Disabled {
        n3415 = local read "Read HUMIDITY"() -> (w4465:string)
        n3416 = Spreadsheet String To Array(delimiter (Tab)=",", format string="", spreadsheet string=w4465, array type (2D Dbl)=string[] []) -> (array=w4484:string[])
        n3417 = for {
          tunnel: w4484 -> [w4493] mode=indexing
          tunnel: string[] ["STATE;", "SET;", "RH;", "T;", "AMB_RH;", "AMB_T;", "PUMP;", "FAN_IN;", "FAN_OUT;", "DEHUM;", "CURRENT;", "STALL;"] -> [w4492] mode=indexing
          tunnel: [w4491] -> w4483 mode=indexing
          n3418 = Match Pattern(string=w4493, regular expression=w4492) -> (after substring=w4491:string)  [unwired: 1 in, 3 out]
        }
        n3419 = Index Array(array=w4483) -> (element #1=→"STATE :":string, element #2=→"SET :":string, element #3=w4473:string, element #4=→"T :":string, element #5=w4471:string, element #6=→"AMB_T :":string, element #7=→"PUMP :":string, element #8=→"FAN_IN :":string, element #9=→"FAN_OUT :":string, element #10=→"DEHUM :":string, element #11=→"CURRENT :":string, element #12=→"STALL :":string)  [unwired: 12 in]
        "RH :" <- w4473
        "AMB_RH :" <- w4471
        n3420 = Fract/Exp String To Number(string=w4473) -> (number=w4466:dbl)  [unwired: 3 in, 1 out]
        n3421 = Fract/Exp String To Number(string=w4471) -> (number=w4470:dbl)  [unwired: 3 in, 1 out]
        n3422 = local write "Ambient Humidity :"(w4470) -> ()
        n3423 = Equal?(x=w4466, y=0.0) -> (x = y?=w4468:bool)
        n3424 = case shown="True" w4468 {
          tunnel: [w4489 w4490] -> w4467
          tunnel: w4466 -> [w4489 _]
          frame False {
            (unwired) 0.0
            "Humidity temp" <- w4489
          }
          frame True {
            n3425 = local read "Humidity temp"() -> (w4490:dbl)
          }
        }
        "RH Numeric:" <- w4467
      }
      frame Enabled {
        n3426 = local read "Read HUMIDITY"() -> (w4516:string)
        n3427 = Spreadsheet String To Array(delimiter (Tab)=",", format string="", spreadsheet string=w4516, array type (2D Dbl)=dbl[] []) -> (array=w4512:dbl[])
        n3428 = Index Array(array=w4512) -> (element #1=→"STATE :":dbl, element #2=→"SET :":dbl, element #3=w4497:dbl, element #4=→"RH :":dbl, element #5=→"T :":dbl, element #6=→"AMB_RH :":dbl, element #7=→"AMB_T :":dbl, element #8=→"PUMP :":dbl, element #9=→"FAN_IN :":dbl, element #10=→"FAN_OUT :":dbl, element #11=→"DEHUM :":dbl, element #12=→"CURRENT :":dbl, element #13=→"STALL":dbl)  [unwired: 13 in]
        "RH Numeric:" <- w4497
        n3429 = Equal?(x=w4497, y=0.0) -> (x = y?=w4500:bool)
        n3430 = case shown="False" w4500 {
          tunnel: [w4517 w4518] -> w4496
          tunnel: w4497 -> [w4517 _]
          frame False {
            "Humidity temp 2" <- w4517
          }
          frame True {
            n3431 = local read "Humidity temp 2"() -> (w4518:dbl)
          }
        }
        n3432 = call <vilib>:"Median Filter PtByPt.vi"("rank"=2, "x"=w4496) -> ("Filtered x"=w4495:dbl)  [unwired: 2 in, 1 out]
      }
    }
    n3433 = local write "RH Numeric:"(w4462) -> ()
    n3434 = local read "Quit"() -> (w4464:bool)
  }
  n3435 = while {
    shift-right: [w4524] -> _
    shift-left: _ -> [w4525]
    shift-right: [w4522] -> _
    shift-left: T20 {"Read Uno"="", "Bytes at Heave Port"=0.0, "UNO COM Port:"="COM9", "UNO COM Port: 2"="COM7", "Residual Due"="", "UNO COM Status 2"=TRUE, "UNO COM Status"=TRUE, "Port 2"=TRUE, "Sway PPR"=6400.0, "Surge PPR"=6400.0, "Heave PPR"=6400.0, "Sway Pitch"=2.0, "Surge Pitch"=3.0, "Heave Pitch"=4.0, "Sway Pulses/mm"=320.0, "Surge Pulses/mm"=1600.0, "Heave Pulses/mm"=1600.0, "inner loop"=0.0, "Read Heave and Surge 2"="", "String 36"="", "Write S"=FALSE, "WriteCC1"=[""], "Heave COM Loop"=0, "LastCom"="", "EXIT"=FALSE, "Error Heave"={"status"=TRUE, "code"=-1073807343, "source"=""}} -> [w4521]
    shift-right: [w4519] -> _
    shift-left: enum16{"init", "MAIN", "Panel Close"}."init" -> [w4520]
    stop <- w4523 stop-if-true
    # "UNO CODE LOGIC"
    n3436 = case shown="\"MAIN\"" w4520 {
      tunnel: w4525 -> [w4539 w4558 w4614 w4616]
      tunnel: [w4534 w4563 w4614 w4616] -> w4524
      tunnel: [_ _ TRUE _] -> w4523
      tunnel: [w4530 w4561 w4612 w4615] -> w4522
      tunnel: w4521 -> [w4536 w4557 w4612 w4615]
      tunnel: [enum16{"init", "MAIN", "Panel Close"}."MAIN" w4552 _ _] -> w4519
      frame "init" {
        n3437 = local read "Com Port 1"() -> (w4526:refnum<visa-resource-name>)
        n3438 = Bundle By Name(cluster=w4536, "UNO COM Port:"=w4526) -> (w4535:T20)
        n3439 = call "Instrument fgv.vi"("Enum"=T32."INIT", "error in (no error) 2"=w4539, "INPUT"=w4535) -> ("error"=w4537:errorcluster, "output"=w4533:T18)  [unwired: 6 in, 1 out]
        n3440 = case shown="Error" w4537 {
          selector: w4537 -> [w4541 _]
          tunnel: [w4541 w4545] -> w4534
          tunnel: w4533 -> [w4540 w4543]
          tunnel: [w4540 w4542] -> w4531
          frame No Error {
          }
          frame Error {
            n3441 = call "Instrument fgv.vi"("Enum"=T32."ERROR INIT", "INPUT"=w4543) -> ("error"=w4546:errorcluster, "output"=w4542:T18)  [unwired: 7 in, 1 out]
            n3442 = call <vilib>:"Clear Errors.vi"("error in (no error)"=w4546) -> ("error out"=w4545:errorcluster)  [unwired: 5 in, 1 out]
          }
        }
        n3443 = local read "LastCom UNO"() -> (w4528:string)
        n3444 = Unbundle By Name(w4531) -> ("Heave COM Status 2"=→"Instrument Status":bool, "Error Heave"=→"Error  2":errorcluster)  [unwired: 1 out]
        n3445 = Bundle By Name(cluster=w4531, "LastCom"=w4528) -> (w4530:T18)
      }
      frame "MAIN" {
        n3446 = Unbundle By Name(w4557) -> ("UNO COM Port: 2"=w4547:refnum<visa-resource-name>)
        n3447 = local read "Com Port 1"() -> (w4548:refnum<visa-resource-name>)
        n3448 = local write "COM Port UNO :"(w4547) -> ()
        n3449 = Equal?(x=w4547, y=w4548) -> (x = y?=w4564:bool)
        n3450 = Bundle By Name(cluster=w4557, "UNO COM Port:"=w4548) -> (w4556:T20)
        n3451 = case shown="True" w4564 {
          tunnel: [w4568 w4585] -> w4563
          tunnel: w4558 -> [w4569 w4591]
          tunnel: w4556 -> [w4567 w4589]
          tunnel: [w4566 w4584] -> w4561
          frame False {
            n3452 = call <vilib>:"Clear Errors.vi"("error in (no error)"=w4569) -> ("error out"=w4565:errorcluster)  [unwired: 5 in, 1 out]
            n3453 = call "Instrument fgv.vi"("Enum"=T32."ERROR INIT", "error in (no error) 2"=w4565, "INPUT"=w4567) -> ("error"=w4571:errorcluster, "output"=w4566:T18)  [unwired: 6 in, 1 out]
            n3454 = call <vilib>:"Clear Errors.vi"("error in (no error)"=w4571) -> ("error out"=w4568:errorcluster)  [unwired: 5 in, 1 out]
          }
          frame True {
            n3455 = call "Instrument fgv.vi"("Enum"=T32."READ", "error in (no error) 2"=w4591, "INPUT"=w4589) -> ("error"=w4590:errorcluster, "output"=w4583:T18)  [unwired: 6 in, 1 out]
            n3456 = Bundle By Name(cluster=w4583, "String 36"="WRITE UNO") -> (w4582:T18)
            n3457 = case shown="True" "Write" {
              selector: "Write" -> [_ w4606]
              tunnel: w4590 -> [w4604 w4611]
              tunnel: [w4604 w4610] -> w4580
              tunnel: w4582 -> [w4603 w4608]
              tunnel: [w4603 w4607] -> w4579
              frame False {
              }
              frame True {
                n3458 = Not(x=w4606) -> (.not. x?=w4605:bool)
                n3459 = local write "Write"(w4605) -> ()
                n3460 = call "Instrument fgv.vi"("Enum"=T32."MANUAL WRITE", "error in (no error) 2"=w4611, "INPUT"=w4608) -> ("error"=w4610:errorcluster, "output"=w4607:T18)  [unwired: 6 in, 1 out]
              }
            }
            n3461 = Array Size(array="Write UNO") -> (size(s)=w4577:i32)
            n3462 = Greater Than 0?(x=w4577) -> (x > 0?=w4576:bool)
            n3463 = call "Instrument fgv.vi"("Enum"=T32."WRITE", "error in (no error) 2"=w4580, "WriteCC1"="Write UNO", "INPUT"=w4579) -> ("error"=w4587:errorcluster, "WriteCC1 2"=w4578:string[], "output"=w4586:T18)  [unwired: 5 in]
            n3464 = case shown="True" w4576 {
              tunnel: w4578 -> [_ w4593]
              frame False {
              }
              frame True {
                n3465 = local write "Write UNO"(w4593) -> ()
              }
            }
            n3466 = case shown="Error" w4587 {
              selector: w4587 -> [w4594 w4597]
              tunnel: w4586 -> [w4595 w4602]
              tunnel: [w4595 w4601] -> w4584
              tunnel: [w4594 w4599] -> w4585
              frame No Error {
              }
              frame Error {
                n3467 = call <vilib>:"Clear Errors.vi"("error in (no error)"=w4597) -> ("error out"=w4596:errorcluster)  [unwired: 5 in, 1 out]
                n3468 = call "Instrument fgv.vi"("Enum"=T32."ERROR INIT", "error in (no error) 2"=w4596, "INPUT"=w4602) -> ("error"=w4600:errorcluster, "output"=w4601:T18)  [unwired: 6 in, 1 out]
                n3469 = call <vilib>:"Clear Errors.vi"("error in (no error)"=w4600) -> ("error out"=w4599:errorcluster)  [unwired: 5 in, 1 out]
              }
            }
            n3470 = Unbundle By Name(w4584) -> ("LastCom"=→"LastCom UNO":string, "Read Heave and Surge"=→"Read UNO":string)
          }
        }
        n3471 = Unbundle By Name(w4561) -> ("Heave COM Status 2"=w4562:bool, "Heave COM Status"=w4551:bool, "Error Heave"=w4549:errorcluster, "Bytes at Heave Port"=→"Bytes at Humidity Port":dbl)
        n3472 = Not(x=w4551) -> (.not. x?=w4559:bool)
        n3473 = Not(x=w4562) -> (.not. x?=w4550:bool)
        n3474 = local write "Instrument Status"(w4559) -> ()
        n3475 = local write "Error  2"(w4549) -> ()
        n3476 = local write "Port 1a"(w4551) -> ()
        n3477 = local read "Quit"() -> (w4553:bool)
        n3478 = local write "COM Status"(w4550) -> ()
        n3479 = Select(t=enum16{"init", "MAIN", "Panel Close"}."Panel Close", s=w4553, f=enum16{"init", "MAIN", "Panel Close"}."MAIN") -> (s? t:f=w4552:enum16{"init", "MAIN", "Panel Close"})
      }
      frame "Panel Close" {
      }
      frame Default {
      }
    }
  }
